vi "FlexMag - 23-03-2023.vi"() -> ()   [LabVIEW 2018] (continued)
            n3949 = local write "CH1_MP_DO"(w6204) -> ()
            n3950 = local write "CH1_TP_BV_DO"(w6207) -> ()
            n3951 = local write "CH1_BG_BV_DO"(w6206) -> ()
            n3952 = local write "CH1_CC_DO"(w6205) -> ()
            n3953 = local write "CH1_Trns_BP_Left_DO"(w6213) -> ()
            n3954 = local write "CH1_SRV1_Piston_For_DO"(w6216) -> ()
            n3955 = local write "CH1_SRV1_Piston_Back_DO"(w6215) -> ()
            n3956 = local write "CH1_WFC_DO"(w6214) -> ()
            n3957 = local read "CH1_PetCool_Down_DI"() -> (w6212:bool)
            n3958 = local read "CH1_Trns_Gv_Open_DI"() -> (w6208:bool)
            n3959 = local read "CH1_Trns_Gv_Close_DI"() -> (w6209:bool)
            n3960 = local read "CH1_Cst_Fix_Down_DI"() -> (w6210:bool)
            n3961 = local read "CH1_PetCool_Up_DI"() -> (w6211:bool)
            n3962 = local read "CH1_TGV_Control_DI"() -> (w6217:bool)
            n3963 = local write "CH1_Trns_Gv_Open_DO"(w6208) -> ()
            n3964 = local write "CH1_Trns_Gv_Close_DO"(w6209) -> ()
            n3965 = local write "CH1_Cst_Fix_DO"(w6210) -> ()
            n3966 = local write "CH1_PetCool_Up_DO"(w6211) -> ()
            n3967 = local write "CH1_PetCool_Down_DO"(w6212) -> ()
            n3968 = local write "CH1_TGV_Control_DO"(w6217) -> ()
          }
        }
      }
      frame #3 {
        # "CH1 DO 1&2"
        n3969 = local read "CH1 I/O Loading"() -> (w6232:bool)
        n3970 = case shown="False" w6232 {
          tunnel: [w6255 w6265] -> w6233
          tunnel: ["CH1_PL_VBV_DO" w6262] -> w6220
          tunnel: ["CH1_CH_VBV_DO" w6262] -> w6219
          frame False {
            n3971 = Build Array("CH1_MP_DO", "CH1_TP_BV_DO", "CH1_BG_BV_DO", "CH1_CH_VBV_DO", "CH1_CH_ATM_DO", "CH1_PL_VBV_DO", "CH1_PL_ATM_DO", "CH1_CC_DO") -> (w6255:bool[])
          }
          frame True {
            w6262 = FALSE
            w6263 = FALSE
            n3972 = local read "CH1_MP_DI"() -> (w6264:bool)
            n3973 = local read "CH1_TP_BV_DI"() -> (w6267:bool)
            n3974 = local read "CH1_BG_BV_DI"() -> (w6268:bool)
            n3975 = local read "CH1_CC_DI"() -> (w6266:bool)
            n3976 = Build Array(w6264, w6267, w6268, w6263, w6263, w6263, w6262, w6266) -> (w6265:bool[])
          }
        }
        "CH1_CH_VBV_DI" <- w6219
        "CH1_PL_VBV_DI" <- w6220
        n3977 = call "MB Serial Master Query Write Multiple Coils (poly).vi"("VISA resource name"=w6224, "Starting Address"=u16 320, "Coils"=w6233, "error in"=w6223, "Serial Parameters"=T15 {"Mode"=enum."RTU", "Slave Address"=1}) -> ("VISA resource name out"=w6229:refnum<visa-resource-name>, "error out"=w6225:errorcluster)  [unwired: 12 in, 1 out]
        n3978 = local read "CH1 I/O Loading"() -> (w6226:bool)
        n3979 = case shown="False" w6226 {
          tunnel: [w6236 w6248] -> w6227
          tunnel: ["CH1_SoV_Ar_DO" w6244] -> w6218
          frame False {
            n3980 = Build Array("CH1_SoV_Ar_DO", "CH1_Trns_Gv_Open_DO", "CH1_Trns_Gv_Close_DO", "CH1_M2_D4_DO", "CH1_Cst_Fix_DO", "CH1_M2_D6_DO", "CH1_PetCool_Up_DO", "CH1_PetCool_Down_DO") -> (w6236:bool[])
          }
          frame True {
            w6244 = FALSE ("element")
            n3981 = local read "CH1_Trns_Gv_Open_DI"() -> (w6252:bool)
            n3982 = local read "CH1_Trns_Gv_Close_DI"() -> (w6251:bool)
            n3983 = local read "CH1_Cst_Fix_Down_DI"() -> (w6247:bool)
            n3984 = local read "CH1_PetCool_Up_DI"() -> (w6246:bool)
            n3985 = local read "CH1_PetCool_Down_DI"() -> (w6245:bool)
            n3986 = local read "CH1_M2_D4_DI"() -> (w6250:bool)
            n3987 = Build Array(w6244, w6252, w6251, w6250, w6247, FALSE ("element"), w6246, w6245) -> (w6248:bool[])
          }
        }
        "CH1_SoV_Ar_DI" <- w6218
        n3988 = call "MB Serial Master Query Write Multiple Coils (poly).vi"("VISA resource name"=w6229, "Starting Address"=u16 320, "Coils"=w6227, "error in"=w6225, "Serial Parameters"=T15 {"Mode"=enum."RTU", "Slave Address"=2}) -> ("VISA resource name out"=w6221:refnum<visa-resource-name>, "error out"=w6222:errorcluster)  [unwired: 12 in, 1 out]
      }
      frame #4 {
        # "CH1 DO 3&4"
        n3989 = local read "CH1 I/O Loading"() -> (w6281:bool)
        n3990 = case shown="False" w6281 {
          tunnel: [w6296 w6306] -> w6280
          frame False {
            n3991 = Build Array("CH1_SRV1_Piston_For_DO", "CH1_SRV1_Piston_Back_DO", "CH1_M3_D3_DO", "CH1_SRV_Direction_Clockwise_DO", "CH1_M3_D5_DO", "CH1_M3_D6_DO", "CH1_WFC_DO", "CH1_Trns_BP_Left_DO") -> (w6296:bool[])
          }
          frame True {
            w6305 = FALSE ("element")
            n3992 = local read "CH1_Trns_BP_Left_DI"() -> (w6307:bool)
            n3993 = local read "CH1_SRV1_Piston_For_DI"() -> (w6308:bool)
            n3994 = local read "CH1_SRV1_Piston_Back_DI"() -> (w6309:bool)
            n3995 = local read "CH1_M3_D6_DI"() -> (w6310:bool)
            n3996 = local read "CH1_WFC_DI"() -> (w6311:bool)
            n3997 = Build Array(w6308, w6309, w6305, w6305, w6305, w6310, w6311, w6307) -> (w6306:bool[])
          }
        }
        n3998 = call "MB Serial Master Query Write Multiple Coils (poly).vi"("VISA resource name"=w6272, "Starting Address"=u16 320, "Coils"=w6280, "error in"=w6271, "Serial Parameters"=T15 {"Mode"=enum."RTU", "Slave Address"=3}) -> ("VISA resource name out"=w6274:refnum<visa-resource-name>, "error out"=w6273:errorcluster)  [unwired: 12 in, 1 out]
        n3999 = local read "CH1 I/O Loading"() -> (w6278:bool)
        n4000 = case shown="False" w6278 {
          tunnel: [w6283 w6292] -> w6275
          frame False {
            n4001 = Build Array("CH1_LN2_DO", "CH1_M4_D2_DO", "CH1_TGV_Control_DO", "CH1_M4_D4_DO", "CH1_Right_Limit_DO", "CH1_Right_Slow_DO", "CH1_M4_D7_DO", "CH1_M4_D8_DO") -> (w6283:bool[])
          }
          frame True {
            w6293 = FALSE ("element")
            w6294 = FALSE ("element")
            n4002 = local read "CH1_TGV_Control_DI"() -> (w6295:bool)
            n4003 = Build Array(w6294, w6294, w6295, w6293, w6293, w6293, w6293, w6293) -> (w6292:bool[])
          }
        }
        n4004 = call "MB Serial Master Query Write Multiple Coils (poly).vi"("VISA resource name"=w6274, "Starting Address"=u16 320, "Coils"=w6275, "error in"=w6273, "Serial Parameters"=T15 {"Mode"=enum."RTU", "Slave Address"=4}) -> ("VISA resource name out"=w6269:refnum<visa-resource-name>, "error out"=w6270:errorcluster)  [unwired: 12 in, 1 out]
      }
      frame #5 {
        # "CH1 AI&AO"
        n4005 = call "MB Serial Master Query Read Input Registers (poly).vi"("VISA resource name"=w6345, "Starting Address"=u16 704 ("Quantity"), "Quantity"=u16 8, "error in"=w6342, "Serial Parameters"=T15 {"Mode"=enum."RTU", "Slave Address"=5}) -> ("VISA resource name out"=w6343:refnum<visa-resource-name>, "Input Registers"=w6333:u16[], "error out"=w6344:errorcluster)  [unwired: 11 in, 1 out]
        n4006 = Index Array(array=w6333, index #1=0 ("index"), index #2=1 ("index"), index #3=2 ("index"), index #4=3 ("index"), index #5=4 ("index"), index #6=5 ("index"), index #7=6 ("index"), index #8=7 ("index")) -> (element #1=→"CH1_Ai_Pl_Pg":u16, element #2=→"CH1_Ai_Ch_Pg":u16, element #3=→"CH1_Ai_Ch_Cc":u16, element #4=→"CH1_Ai_A4":u16, element #5=→"CH1_Ai_A5":u16, element #6=→"CH1_Ai_A6":u16, element #7=→"CH1_LN2_TK_t":u16, element #8=→"CH1_LN2_TK_b":u16)
        n4007 = Build Array(FALSE, "CH1 MW1 Set", "CH1 MW2 Set", "CH1 AO3 Set", "CH1 AO4 Set") -> (w6317:bool[])
        n4008 = Boolean Array To Number(Boolean array=w6317) -> (number=w6316:u32)
        n4009 = Mantissa & Exponent(0:w6316) -> (2:w6315:dbl)  [unwired: 1 out]
        n4010 = case shown="1" w6315 {
          tunnel: [0.0 ("TC2_Set_Value") "CH1 MW1" "CH1 MW2" "CH1 AO3" "CH1 AO4"] -> w6313
          tunnel: [0 1184 1185 1186 1187] -> w6314
          frame 0, Default {
          }
          frame 1 {
            n4011 = local write "CH1 MW1 Set"(FALSE ("CH1 AO1 Set")) -> ()
          }
          frame 2 {
            n4012 = local write "CH1 MW2 Set"(FALSE ("CH1 AO2 Set")) -> ()
          }
          frame 3 {
            n4013 = local write "CH1 AO3 Set"(FALSE ("CH1 AO3 Set")) -> ()
          }
          frame 4 {
            n4014 = local write "CH1 AO4 Set"(FALSE ("CH1 AO4 Set")) -> ()
          }
        }
        n4015 = Build Array(w6313) -> (w6312:dbl[])
        n4016 = call "MB Serial Master Query Write Multiple Registers (poly).vi"("VISA resource name"=w6343, "Starting Address"=w6314, "Registers"=w6312, "error in"=w6344, "Serial Parameters"=T15 {"Mode"=enum."RTU", "Slave Address"=6}) -> ("VISA resource name out"=w6348:refnum<visa-resource-name>, "error out"=w6347:errorcluster)  [unwired: 12 in, 1 out]
      }
      frame #6 {
      }
      frame #7 {
      }
    }
  }
  n4017 = while {
    tunnel: w119 -> [w6370]
    tunnel: w120 -> [w6369]
    tunnel: [w6365] -> w121
    tunnel: [w6364] -> w122
    i -> [w6366]
    stop <- FALSE stop-if-true
    n4018 = Wait Until Next ms Multiple(millisecond multiple=u32 300) -> ()  [unwired: 1 out]
    n4019 = Less Or Equal?(x=w6366, y=5) -> (x <= y?=→"CH3 I/O Loading":bool)
    n4020 = stacked-sequence {
      seq-local: [w6373 _ _ _ _ _ _ _] -> [_ w6422 _ _ _ _ _ _]
      seq-local: [w6374 _ _ _ _ _ _ _] -> [_ w6421 _ _ _ _ _ _]
      seq-local: [_ w6419 _ _ _ _ _ _] -> [_ _ _ w6488 _ _ _ _]
      seq-local: [_ _ _ w6485 _ _ _ _] -> [_ _ _ _ w6536 _ _ _]
      seq-local: [_ _ _ _ w6534 _ _ _] -> [_ _ _ _ _ w6593 _ _]
      seq-local: [_ _ _ w6486 _ _ _ _] -> [_ _ _ _ w6533 _ _ _]
      seq-local: [_ w6420 _ _ _ _ _ _] -> [_ _ _ w6487 _ _ _ _]
      seq-local: [_ _ _ _ w6535 _ _ _] -> [_ _ _ _ _ w6594 _ _]
      tunnel: w6370 -> [w6376 _ _ _ _ _ _ _]
      tunnel: w6369 -> [w6375 _ _ _ _ _ _ _]
      tunnel: [_ _ _ _ _ w6590 _ _] -> w6365
      tunnel: [_ _ _ _ _ w6589 _ _] -> w6364
      frame #0 {
        # "CH3 DI 1&2"
        n4021 = call "MB Serial Master Query Read Discrete Inputs (poly).vi"("VISA resource name"=w6376, "Starting Address"=u16 0 ("Quantity"), "Quantity"=u16 8, "error in"=w6375, "Serial Parameters"=T15 {"Mode"=enum."RTU", "Slave Address"=1}) -> ("VISA resource name out"=w6409:refnum<visa-resource-name>, "Discrete Inputs"=w6393:bool[], "error out"=w6408:errorcluster)  [unwired: 11 in, 1 out]
        n4022 = Index Array(array=w6393, index #1=0 ("index"), index #2=1 ("index"), index #3=2 ("index"), index #4=3 ("index"), index #5=4 ("index"), index #6=5 ("index"), index #7=6 ("index"), index #8=7 ("index")) -> (element #1=→"CH3_MP_DI":bool, element #2=→"CH3_TP_BV_DI":bool, element #3=→"CH3_BG_BV_DI":bool, element #5=→"CH3_CH_ATM_DI":bool, element #7=→"CH3_PL_ATM_DI":bool, element #8=→"CH3_CC_DI":bool)  [unwired: 2 out]
        n4023 = call "MB Serial Master Query Read Discrete Inputs (poly).vi"("VISA resource name"=w6409, "Starting Address"=u16 0 ("Quantity"), "Quantity"=u16 8, "error in"=w6408, "Serial Parameters"=T15 {"Mode"=enum."RTU", "Slave Address"=2}) -> ("VISA resource name out"=w6373:refnum<visa-resource-name>, "Discrete Inputs"=w6377:bool[], "error out"=w6374:errorcluster)  [unwired: 11 in, 1 out]
        n4024 = Index Array(array=w6377, index #1=0 ("index"), index #2=1 ("index"), index #3=2 ("index"), index #4=3 ("index"), index #5=4 ("index"), index #6=5 ("index"), index #7=6 ("index"), index #8=7 ("index")) -> (element #2=→"CH3_Trns_Gv_Open_DI":bool, element #3=→"CH3_Trns_Gv_Close_DI":bool, element #4=→"CH3_Trns_BP_Right_DI":bool, element #5=→"CH3_Cst_Fix_Up_DI":bool, element #6=→"CH3_Cst_Fix_Down_DI":bool, element #7=→"CH3_PetCool_Up_DI":bool, element #8=→"CH3_PetCool_Down_DI":bool)  [unwired: 1 out]
      }
      frame #1 {
        # "CH3 DI 3&4"
        n4025 = call "MB Serial Master Query Read Discrete Inputs (poly).vi"("VISA resource name"=w6422, "Starting Address"=u16 0 ("Quantity"), "Quantity"=u16 8, "error in"=w6421, "Serial Parameters"=T15 {"Mode"=enum."RTU", "Slave Address"=3}) -> ("VISA resource name out"=w6457:refnum<visa-resource-name>, "Discrete Inputs"=w6440:bool[], "error out"=w6456:errorcluster)  [unwired: 11 in, 1 out]
        n4026 = local read "water bypass"() -> (w6418:bool)
        n4027 = Index Array(array=w6440, index #1=0 ("index"), index #2=1 ("index"), index #3=2 ("index"), index #4=3 ("index"), index #5=4 ("index"), index #6=5 ("index"), index #7=6 ("index"), index #8=7 ("index")) -> (element #1=→"CH3_SRV1_Piston_For_DI":bool, element #2=→"CH3_SRV1_Piston_Back_DI":bool, element #3=→"CH3_SRV_Start_Stop_DI":bool, element #4=→"CH3_SRV_Left_Direction_DI3":bool, element #5=→"CH3_SRV2_COUNTER_DI":bool, element #6=→"CH3_M3_D6_DI":bool, element #7=w6416:bool, element #8=→"CH3_Trns_BP_Left_DI":bool)
        n4028 = case shown="True" w6418 {
          tunnel: w6416 -> [w6464 _]
          tunnel: [w6464 w6465] -> w6417
          frame False {
          }
          frame True {
            n4029 = local read "CH3_WFC_DO"() -> (w6465:bool)
          }
        }
        "CH3_WFC_DI" <- w6417
        n4030 = call "MB Serial Master Query Read Discrete Inputs (poly).vi"("VISA resource name"=w6457, "Starting Address"=u16 0 ("Quantity"), "Quantity"=u16 8, "error in"=w6456, "Serial Parameters"=T15 {"Mode"=enum."RTU", "Slave Address"=4}) -> ("VISA resource name out"=w6419:refnum<visa-resource-name>, "Discrete Inputs"=w6423:bool[], "error out"=w6420:errorcluster)  [unwired: 11 in, 1 out]
        n4031 = Index Array(array=w6423, index #1=0 ("index"), index #2=1 ("index"), index #3=2 ("index"), index #4=3 ("index"), index #5=4 ("index"), index #6=5 ("index"), index #7=6 ("index"), index #8=7 ("index")) -> (element #1=→"CH3_Air_Pressure_DI":bool, element #2=→"CH3_DS_DI":bool, element #3=→"CH3_TGV_Control_DI":bool, element #4=→"CH3_Trns_Interlock_DI":bool, element #5=→"CH3_Right_Limit_DI":bool, element #6=→"CH3_Right_Slow_DI":bool, element #7=→"CH3_Left_Slow_DI":bool, element #8=→"CH3_Left_Limit_DI":bool)
      }
      frame #2 {
        n4032 = local read "CH3 I/O Loading"() -> (w6466:bool)
        n4033 = case shown="True" w6466 {
          frame False {
          }
          frame True {
            n4034 = local read "CH3_SRV1_Piston_Back_DI"() -> (w6470:bool)
            n4035 = local read "CH3_SRV1_Piston_For_DI"() -> (w6471:bool)
            n4036 = local read "CH3_Trns_BP_Left_DI"() -> (w6468:bool)
            n4037 = local read "CH3_BG_BV_DI"() -> (w6473:bool)
            n4038 = local read "CH3_TP_BV_DI"() -> (w6474:bool)
            n4039 = local read "CH3_WFC_DI"() -> (w6469:bool)
            n4040 = local read "CH3_MP_DI"() -> (w6475:bool)
            n4041 = local read "CH3_CC_DI"() -> (w6472:bool)
            n4042 = local write "CH3_MP_DO"(w6475) -> ()
            n4043 = local write "CH3_TP_BV_DO"(w6474) -> ()
            n4044 = local write "CH3_BG_BV_DO"(w6473) -> ()
            n4045 = local write "CH3_CC_DO"(w6472) -> ()
            n4046 = local write "CH3_Trns_BP_Left_DO"(w6468) -> ()
            n4047 = local write "CH3_SRV1_Piston_For_DO"(w6471) -> ()
            n4048 = local write "CH3_SRV1_Piston_Back_DO"(w6470) -> ()
            n4049 = local write "CH3_WFC_DO"(w6469) -> ()
            n4050 = local read "CH3_PetCool_Down_DI"() -> (w6481:bool)
            n4051 = local read "CH3_Trns_Gv_Open_DI"() -> (w6476:bool)
            n4052 = local read "CH3_Trns_Gv_Close_DI"() -> (w6477:bool)
            n4053 = local read "CH3_Cst_Fix_Down_DI"() -> (w6479:bool)
            n4054 = local read "CH3_Trns_BP_Right_DI"() -> (w6478:bool)
            n4055 = local read "CH3_PetCool_Up_DI"() -> (w6480:bool)
            n4056 = local read "CH3_TGV_Control_DI"() -> (w6467:bool)
            n4057 = local write "CH3_Trns_BP_Right_DO"(w6478) -> ()
            n4058 = local write "CH3_Trns_GV_Open_DO"(w6476) -> ()
            n4059 = local write "CH3_Trns_GV_Close_DO"(w6477) -> ()
            n4060 = local write "CH3_Cst_Fix_DO"(w6479) -> ()
            n4061 = local write "CH3_PetCool_Up_DO"(w6480) -> ()
            n4062 = local write "CH3_PetCool_Down_DO"(w6481) -> ()
            n4063 = local write "CH3_TGV_Control_DO"(w6467) -> ()
          }
        }
      }
      frame #3 {
        # "CH3 DO 1&2"
        n4064 = local read "CH3 I/O Loading"() -> (w6490:bool)
        n4065 = case shown="False" w6490 {
          tunnel: [w6519 w6532] -> w6492
          tunnel: ["CH3_PL_VBV_DO" w6527] -> w6484
          tunnel: ["CH3_CH_VBV_DO" w6527] -> w6483
          frame False {
            n4066 = Build Array("CH3_MP_DO", "CH3_TP_BV_DO", "CH3_BG_BV_DO", "CH3_CH_VBV_DO", "CH3_CH_ATM_DO", "CH3_PL_VBV_DO", "CH3_PL_ATM_DO", "CH3_CC_DO") -> (w6519:bool[])
          }
          frame True {
            w6527 = FALSE
            w6526 = FALSE
            n4067 = local read "CH3_CC_DI"() -> (w6528:bool)
            n4068 = local read "CH3_BG_BV_DI"() -> (w6529:bool)
            n4069 = local read "CH3_TP_BV_DI"() -> (w6531:bool)
            n4070 = local read "CH3_MP_DI"() -> (w6530:bool)
            n4071 = Build Array(w6530, w6531, w6529, w6526, w6526, w6526, w6527, w6528) -> (w6532:bool[])
          }
        }
        "CH3_CH_VBV_DI" <- w6483
        "CH3_PL_VBV_DI" <- w6484
        n4072 = call "MB Serial Master Query Write Multiple Coils (poly).vi"("VISA resource name"=w6488, "Starting Address"=u16 320, "Coils"=w6492, "error in"=w6487, "Serial Parameters"=T15 {"Mode"=enum."RTU", "Slave Address"=1}) -> ("VISA resource name out"=w6494:refnum<visa-resource-name>, "error out"=w6493:errorcluster)  [unwired: 12 in, 1 out]
        n4073 = local read "CH3 I/O Loading"() -> (w6489:bool)
        n4074 = case shown="False" w6489 {
          tunnel: [w6500 w6516] -> w6491
          tunnel: ["CH3_SoV_Ar_DO" w6508] -> w6482
          frame False {
            n4075 = Build Array("CH3_SoV_Ar_DO", "CH3_Trns_GV_Open_DO", "CH3_Trns_GV_Close_DO", "CH3_Trns_BP_Right_DO", "CH3_Cst_Fix_DO", "CH3_M2_D6_DO", "CH3_PetCool_Up_DO", "CH3_PetCool_Down_DO") -> (w6500:bool[])
          }
          frame True {
            w6508 = FALSE
            n4076 = local read "CH3_PetCool_Down_DI"() -> (w6514:bool)
            n4077 = local read "CH3_Trns_Gv_Open_DI"() -> (w6515:bool)
            n4078 = local read "CH3_Trns_Gv_Close_DI"() -> (w6510:bool)
            n4079 = local read "CH3_Trns_BP_Right_DI"() -> (w6511:bool)
            n4080 = local read "CH3_Cst_Fix_Down_DI"() -> (w6512:bool)
            n4081 = local read "CH3_PetCool_Up_DI"() -> (w6513:bool)
            n4082 = Build Array(w6508, w6515, w6510, w6511, w6512, FALSE ("element"), w6513, w6514) -> (w6516:bool[])
          }
        }
        "CH3_SoV_Ar_DI" <- w6482
        n4083 = call "MB Serial Master Query Write Multiple Coils (poly).vi"("VISA resource name"=w6494, "Starting Address"=u16 320, "Coils"=w6491, "error in"=w6493, "Serial Parameters"=T15 {"Mode"=enum."RTU", "Slave Address"=2}) -> ("VISA resource name out"=w6485:refnum<visa-resource-name>, "error out"=w6486:errorcluster)  [unwired: 12 in, 1 out]
      }
      frame #4 {
        # "CH3 DO 3&4"
        n4084 = local read "CH3 I/O Loading"() -> (w6538:bool)
        n4085 = case shown="False" w6538 {
          tunnel: [w6560 w6575] -> w6539
          frame False {
            n4086 = Build Array("CH3_SRV1_Piston_For_DO", "CH3_SRV1_Piston_Back_DO", "CH3_M3_D3_DO", "CH3_SRV_Direction_Clockwise_DO", "CH3_M3_D5_DO", "CH3_M3_D6_DO", "CH3_WFC_DO", "CH3_Trns_BP_Left_DO") -> (w6560:bool[])
          }
          frame True {
            w6569 = FALSE
            n4087 = local read "CH3_SRV1_Piston_Back_DI"() -> (w6573:bool)
            n4088 = local read "CH3_SRV1_Piston_For_DI"() -> (w6574:bool)
            n4089 = local read "CH3_Trns_BP_Left_DI"() -> (w6570:bool)
            n4090 = local read "CH3_M3_D6_DI"() -> (w6572:bool)
            n4091 = local read "CH3_WFC_DI"() -> (w6571:bool)
            n4092 = Build Array(w6574, w6573, w6569, w6569, w6569, w6572, w6571, w6570) -> (w6575:bool[])
          }
        }
        n4093 = call "MB Serial Master Query Write Multiple Coils (poly).vi"("VISA resource name"=w6536, "Starting Address"=u16 320, "Coils"=w6539, "error in"=w6533, "Serial Parameters"=T15 {"Mode"=enum."RTU", "Slave Address"=3}) -> ("VISA resource name out"=w6542:refnum<visa-resource-name>, "error out"=w6541:errorcluster)  [unwired: 12 in, 1 out]
        n4094 = local read "CH3 I/O Loading"() -> (w6537:bool)
        n4095 = case shown="False" w6537 {
          tunnel: [w6547 w6557] -> w6540
          frame False {
            n4096 = Build Array("CH3_LN2_DO", "CH3_M4_D2_DO", "CH3_TGV_Control_DO", "CH3_M4_D4_DO", "CH3_Right_Limit_DO", "CH3_Right_Slow_DO", "CH3_Left_Slow_DO", "CH3_Left_Limit_DO") -> (w6547:bool[])
          }
          frame True {
            w6559 = FALSE
            w6558 = FALSE
            n4097 = local read "CH3_TGV_Control_DI"() -> (w6556:bool)
            n4098 = Build Array(w6558, w6558, w6556, w6559, w6559, w6559, w6559, w6559) -> (w6557:bool[])
          }
        }
        n4099 = call "MB Serial Master Query Write Multiple Coils (poly).vi"("VISA resource name"=w6542, "Starting Address"=u16 320, "Coils"=w6540, "error in"=w6541, "Serial Parameters"=T15 {"Mode"=enum."RTU", "Slave Address"=4}) -> ("VISA resource name out"=w6535:refnum<visa-resource-name>, "error out"=w6534:errorcluster)  [unwired: 12 in, 1 out]
      }
      frame #5 {
        # "CH3 AI&AO"
        n4100 = call "MB Serial Master Query Read Input Registers (poly).vi"("VISA resource name"=w6594, "Starting Address"=u16 704, "Quantity"=u16 8, "error in"=w6593, "Serial Parameters"=T15 {"Mode"=enum."RTU", "Slave Address"=5}) -> ("VISA resource name out"=w6592:refnum<visa-resource-name>, "Input Registers"=w6605:u16[], "error out"=w6591:errorcluster)  [unwired: 11 in, 1 out]
        n4101 = Index Array(array=w6605, index #1=0 ("index"), index #2=1 ("index"), index #3=2 ("index"), index #4=3 ("index"), index #5=4 ("index"), index #6=5 ("index"), index #7=6 ("index"), index #8=7 ("index")) -> (element #1=→"CH3_Ai_Pl_Pg":u16, element #2=→"CH3_Ai_Ch_Pg":u16, element #3=→"CH3_Ai_Ch_Cc":u16, element #4=→"MFC_Ar_Read_value":u16, element #5=→"CH3_Ai_A5":u16, element #6=→"CH3_Ai_A6":u16, element #7=→"CH3_LN2_TK_t":u16, element #8=→"CH3_LN2_TK_b":u16)
        n4102 = Build Array(FALSE, "CH3 AO1 Set", "CH3 AO2 Set", "CH3 AO3 Set", "MFC_Ar_Set") -> (w6581:bool[])
        n4103 = Boolean Array To Number(Boolean array=w6581) -> (number=w6580:u32)
        n4104 = Mantissa & Exponent(0:w6580) -> (2:w6579:dbl)  [unwired: 1 out]
        n4105 = case shown="4" w6579 {
          tunnel: [0.0 ("TC2_Set_Value") "CH3 AO1" "CH3 AO2" "CH3 AO3" w6628] -> w6577
          tunnel: [0 1184 1185 1186 1187] -> w6578
          frame 0, Default {
          }
          frame 1 {
            n4106 = local write "CH3 AO1 Set"(FALSE ("CH1 AO1 Set")) -> ()
          }
          frame 2 {
            n4107 = local write "CH3 AO2 Set"(FALSE ("CH1 AO2 Set")) -> ()
          }
          frame 3 {
            n4108 = local write "CH3 AO3 Set"(FALSE ("CH1 AO3 Set")) -> ()
          }
          frame 4 {
            n4109 = local write "MFC_Ar_Set"(FALSE ("CH2 AO4 Set")) -> ()
            n4110 = Divide(x=2048.0, y=200.0) -> (x/y=w6630:dbl)
            n4111 = Multiply(x="MFC_Ar_Set_value", y=w6630) -> (x*y=w6627:dbl)
            n4112 = In Range and Coerce(upper limit=2048.0, x=w6627, lower limit=0.0) -> (coerced(x)=w6628:dbl)  [unwired: 1 out]
          }
        }
        n4113 = Build Array(w6577) -> (w6576:dbl[])
        n4114 = call "MB Serial Master Query Write Multiple Registers (poly).vi"("VISA resource name"=w6592, "Starting Address"=w6578, "Registers"=w6576, "error in"=w6591, "Serial Parameters"=T15 {"Mode"=enum."RTU", "Slave Address"=6}) -> ("VISA resource name out"=w6590:refnum<visa-resource-name>, "error out"=w6589:errorcluster)  [unwired: 12 in, 1 out]
      }
      frame #6 {
      }
      frame #7 {
      }
    }
  }
  n4115 = while {
    tunnel: w144 -> [w6641]
    tunnel: w143 -> [w6640]
    tunnel: [w6639] -> w142
    tunnel: [w6638] -> w141
    i -> [w6637]
    stop <- FALSE stop-if-true
    n4116 = Wait Until Next ms Multiple(millisecond multiple=u32 300) -> ()  [unwired: 1 out]
    n4117 = Less Or Equal?(x=w6637, y=5) -> (x <= y?=→"Center I/O Loading":bool)
    n4118 = stacked-sequence {
      seq-local: [w6647 _ _] -> [_ w6692 _]
      seq-local: [w6646 _ _] -> [_ w6691 _]
      seq-local: [_ w6693 _] -> [_ _ w6745]
      seq-local: [_ w6690 _] -> [_ _ w6744]
      tunnel: w6641 -> [w6648 _ _]
      tunnel: w6640 -> [w6645 _ _]
      tunnel: [_ _ w6743] -> w6639
      tunnel: [_ _ w6742] -> w6638
      frame #0 {
        # "Digital Inputs"
        n4119 = call "MB Serial Master Query Read Discrete Inputs (poly).vi"("VISA resource name"=w6648, "Starting Address"=u16 0 ("Quantity"), "Quantity"=u16 8, "error in"=w6645, "Serial Parameters"=T15 {"Mode"=enum."RTU", "Slave Address"=1}) -> ("VISA resource name out"=w6667:refnum<visa-resource-name>, "Discrete Inputs"=w6683:bool[], "error out"=w6666:errorcluster)  [unwired: 11 in, 1 out]
        n4120 = Index Array(array=w6683, index #1=0 ("index"), index #2=1 ("index"), index #3=2 ("index"), index #4=3 ("index"), index #5=4 ("index"), index #6=5 ("index"), index #7=6 ("index"), index #8=7 ("index")) -> (element #1=→"Casette_Servo_Start/Stop DI":bool, element #2=→"Casette_Servo_Left_Direction DI":bool, element #3=→"Tension_Controllers_Start/Stop DI":bool, element #4=→"Cnt_Right_Limit DI":bool, element #5=→"Cnt_Right_Slow DI":bool, element #6=→"Cnt_Left_Slow DI":bool, element #7=→"Cnt_Left_Limit DI":bool, element #8=→"WFC DI":bool)
        n4121 = call "MB Serial Master Query Read Discrete Inputs (poly).vi"("VISA resource name"=w6667, "Starting Address"=u16 0 ("Quantity"), "Quantity"=u16 8, "error in"=w6666, "Serial Parameters"=T15 {"Mode"=enum."RTU", "Slave Address"=2}) -> ("VISA resource name out"=w6647:refnum<visa-resource-name>, "Discrete Inputs"=w6657:bool[], "error out"=w6646:errorcluster)  [unwired: 11 in, 1 out]
        n4122 = Index Array(array=w6657, index #1=0 ("index"), index #2=1 ("index"), index #3=2 ("index"), index #4=3 ("index"), index #5=4 ("index"), index #6=5 ("index"), index #7=6 ("index"), index #8=7 ("index")) -> (element #1=→"DCPS_ SW1 DI":bool, element #2=→"DCPS_ SW2 DI":bool, element #3=→"DCPS_ SW3 DI":bool, element #4=→"DCPS_ SW4 DI":bool, element #5=→"MW1 DI":bool, element #6=→"MW2 DI":bool, element #7=→"Center_2 DI7":bool, element #8=→"Center_2 DI8":bool)
      }
      frame #1 {
        # "Digital Outputs"
        n4123 = local read "Center I/O Loading"() -> (w6695:bool)
        n4124 = case shown="False" w6695 {
          tunnel: [w6722 w6731] -> w6702
          frame False {
            n4125 = Build Array("Casette_Servo_Start/Stop DO", "Casette_Servo_Left_Direction DO", "Tension_Controllers_Start/Stop DO", "Cnt_Right_Limit DO", "Cnt_Right_Slow DO", "Cnt_Left_Slow DO", "Cnt_Left_Limit DO", "Buzzer DO") -> (w6722:bool[])
          }
          frame True {
            n4126 = local read "Tension_Controllers_Start/Stop DI"() -> (w6737:bool)
            n4127 = local read "Casette_Servo_Left_Direction DI"() -> (w6738:bool)
            n4128 = local read "Casette_Servo_Start/Stop DI"() -> (w6739:bool)
            n4129 = local read "Cnt_Right_Limit DI"() -> (w6736:bool)
            n4130 = local read "Cnt_Right_Slow DI"() -> (w6735:bool)
            n4131 = local read "Cnt_Left_Slow DI"() -> (w6734:bool)
            n4132 = local read "Cnt_Left_Limit DI"() -> (w6733:bool)
            n4133 = Build Array(w6739, w6738, w6737, w6736, w6735, w6734, w6733, FALSE ("element")) -> (w6731:bool[])
          }
        }
        n4134 = call "MB Serial Master Query Write Multiple Coils (poly).vi"("VISA resource name"=w6692, "Starting Address"=u16 320, "Coils"=w6702, "error in"=w6691, "Serial Parameters"=T15 {"Mode"=enum."RTU", "Slave Address"=1}) -> ("VISA resource name out"=w6697:refnum<visa-resource-name>, "error out"=w6696:errorcluster)  [unwired: 12 in, 1 out]
        n4135 = local read "Center I/O Loading"() -> (w6694:bool)
        n4136 = case shown="True" w6694 {
          tunnel: [w6712 w6717] -> w6699
          frame False {
            n4137 = Build Array("DCPS_ SW1 DO", "DCPS_ SW2 DO", "DCPS_ SW3  DO", "DCPS_ SW4 DO", "Center_2 DO5", "Center_2 DO6", "Center_2 DO7", "Center_2 DO8") -> (w6712:bool[])
          }
          frame True {
            n4138 = local read "DCPS_ SW3 DI"() -> (w6719:bool)
            n4139 = local read "DCPS_ SW2 DI"() -> (w6720:bool)
            n4140 = local read "DCPS_ SW4 DI"() -> (w6718:bool)
            n4141 = local read "DCPS_ SW1 DI"() -> (w6721:bool)
            n4142 = Build Array(w6721, w6720, w6719, w6718, FALSE ("element"), FALSE ("element"), FALSE ("element"), FALSE ("element")) -> (w6717:bool[])
          }
        }
        n4143 = call "MB Serial Master Query Write Multiple Coils (poly).vi"("VISA resource name"=w6697, "Starting Address"=u16 320, "Coils"=w6699, "error in"=w6696, "Serial Parameters"=T15 {"Mode"=enum."RTU", "Slave Address"=2}) -> ("VISA resource name out"=w6693:refnum<visa-resource-name>, "error out"=w6690:errorcluster)  [unwired: 12 in, 1 out]
      }
      frame #2 {
        # "Analog Outputs"
        n4144 = Build Array(FALSE, "Center AO1 Set", "Cassette_Servo_Speed Set", "TC1 Set moxa", "TC2 Set moxa") -> (w6754:bool[])
        n4145 = Boolean Array To Number(Boolean array=w6754) -> (number=w6755:u32)
        n4146 = Mantissa & Exponent(0:w6755) -> (2:w6749:dbl)  [unwired: 1 out]
        n4147 = case shown="2" w6749 {
          tunnel: [0.0 ("TC2_Set_Value") "Center AO1" "Cassette_Servo_Speed AO" w6764 w6772] -> w6748
          tunnel: [0 1184 1185 1186 1187] -> w6746
          frame 0, Default {
          }
          frame 1 {
            n4148 = local write "Center AO1 Set"(FALSE ("Center AO1 Set")) -> ()
          }
          frame 2 {
            n4149 = local write "Cassette_Servo_Speed Set"(FALSE ("Center AO2 Set")) -> ()
          }
          frame 3 {
            n4150 = local write "TC1 Set moxa"(FALSE ("TC1 Set")) -> ()
            n4151 = Divide(x=4096.0, y=10.0) -> (x/y=w6768:dbl)
            n4152 = Multiply(x=w6768, y="TC1_Set_Value_Moxa") -> (x*y=w6764:dbl)
          }
          frame 4 {
            n4153 = local write "TC2 Set moxa"(FALSE ("TC2 Set")) -> ()
            n4154 = Divide(x=4096.0, y=10.0) -> (x/y=w6775:dbl)
            n4155 = Multiply(x=w6775, y="TC2_Set_Value_Moxa") -> (x*y=w6772:dbl)
          }
        }
        n4156 = Build Array(w6748) -> (w6747:dbl[])
        n4157 = call "MB Serial Master Query Write Multiple Registers (poly).vi"("VISA resource name"=w6745, "Starting Address"=w6746, "Registers"=w6747, "error in"=w6744, "Serial Parameters"=T15 {"Mode"=enum."RTU", "Slave Address"=3}) -> ("VISA resource name out"=w6743:refnum<visa-resource-name>, "error out"=w6742:errorcluster)  [unwired: 12 in, 1 out]
      }
    }
  }
  n4158 = while {
    tunnel: w126 -> [w6784]
    tunnel: w125 -> [w6783]
    tunnel: [w6779] -> w124
    tunnel: [w6778] -> w123
    i -> [w6780]
    stop <- FALSE stop-if-true
    n4159 = Wait Until Next ms Multiple(millisecond multiple=u32 300) -> ()  [unwired: 1 out]
    n4160 = Less Or Equal?(x=w6780, y=5) -> (x <= y?=→"CH2 I/O Loading":bool)
    n4161 = stacked-sequence {
      seq-local: [w6789 _ _ _ _ _ _ _] -> [_ w6836 _ _ _ _ _ _]
      seq-local: [w6788 _ _ _ _ _ _ _] -> [_ w6834 _ _ _ _ _ _]
      seq-local: [_ w6835 _ _ _ _ _ _] -> [_ _ _ w6902 _ _ _ _]
      seq-local: [_ _ _ w6899 _ _ _ _] -> [_ _ _ _ w6951 _ _ _]
      seq-local: [_ _ _ _ w6949 _ _ _] -> [_ _ _ _ _ w7009 _ _]
      seq-local: [_ _ _ w6900 _ _ _ _] -> [_ _ _ _ w6950 _ _ _]
      seq-local: [_ w6833 _ _ _ _ _ _] -> [_ _ _ w6901 _ _ _ _]
      seq-local: [_ _ _ _ w6948 _ _ _] -> [_ _ _ _ _ w7010 _ _]
      tunnel: w6784 -> [w6790 _ _ _ _ _ _ _]
      tunnel: w6783 -> [w6787 _ _ _ _ _ _ _]
      tunnel: [_ _ _ _ _ w7006 _ _] -> w6779
      tunnel: [_ _ _ _ _ w7005 _ _] -> w6778
      frame #0 {
        # "CH2 DI 1&2"
        n4162 = call "MB Serial Master Query Read Discrete Inputs (poly).vi"("VISA resource name"=w6790, "Starting Address"=u16 0 ("Quantity"), "Quantity"=u16 8, "error in"=w6787, "Serial Parameters"=T15 {"Mode"=enum."RTU", "Slave Address"=1}) -> ("VISA resource name out"=w6823:refnum<visa-resource-name>, "Discrete Inputs"=w6807:bool[], "error out"=w6822:errorcluster)  [unwired: 11 in, 1 out]
        n4163 = Index Array(array=w6807, index #1=0 ("index"), index #2=1 ("index"), index #3=2 ("index"), index #4=3 ("index"), index #5=4 ("index"), index #6=5 ("index"), index #7=6 ("index"), index #8=7 ("index")) -> (element #1=→"CH2_MP_DI":bool, element #2=→"CH2_TP_BV_DI":bool, element #3=→"CH2_BG_BV_DI":bool, element #5=→"CH2_CH_ATM_DI":bool, element #7=→"CH2_PL_ATM_DI":bool, element #8=→"CH2_CC_DI":bool)  [unwired: 2 out]
        n4164 = call "MB Serial Master Query Read Discrete Inputs (poly).vi"("VISA resource name"=w6823, "Starting Address"=u16 0 ("Quantity"), "Quantity"=u16 8, "error in"=w6822, "Serial Parameters"=T15 {"Mode"=enum."RTU", "Slave Address"=2}) -> ("VISA resource name out"=w6789:refnum<visa-resource-name>, "Discrete Inputs"=w6791:bool[], "error out"=w6788:errorcluster)  [unwired: 11 in, 1 out]
        n4165 = Index Array(array=w6791, index #1=0 ("index"), index #2=1 ("index"), index #3=2 ("index"), index #4=3 ("index"), index #5=4 ("index"), index #6=5 ("index"), index #7=6 ("index"), index #8=7 ("index")) -> (element #2=→"CH2_Trns_Gv_Open_DI":bool, element #3=→"CH2_Trns_Gv_Close_DI":bool, element #4=→"CH2_Trns_BP_Right_DI":bool, element #5=→"CH2_Cst_Fix_Up_DI":bool, element #6=→"CH2_Cst_Fix_Down_DI":bool, element #7=→"CH2_PetCool_Up_DI":bool, element #8=→"CH2_PetCool_Down_DI":bool)  [unwired: 1 out]
      }
      frame #1 {
        n4166 = call "MB Serial Master Query Read Discrete Inputs (poly).vi"("VISA resource name"=w6836, "Starting Address"=u16 0 ("Quantity"), "Quantity"=u16 8, "error in"=w6834, "Serial Parameters"=T15 {"Mode"=enum."RTU", "Slave Address"=3}) -> ("VISA resource name out"=w6871:refnum<visa-resource-name>, "Discrete Inputs"=w6837:bool[], "error out"=w6870:errorcluster)  [unwired: 11 in, 1 out]
        n4167 = local read "water bypass"() -> (w6832:bool)
        n4168 = Index Array(array=w6837, index #1=0 ("index"), index #2=1 ("index"), index #3=2 ("index"), index #4=3 ("index"), index #5=4 ("index"), index #6=5 ("index"), index #7=6 ("index"), index #8=7 ("index")) -> (element #1=→"CH2_SRV1_Piston_For_DI":bool, element #2=→"CH2_SRV1_Piston_Back_DI":bool, element #3=→"CH2_SRV_Start_Stop_DI":bool, element #4=→"CH2_SRV_Left_Direction_DI":bool, element #5=→"CH2_SRV2_COUNTER_DI":bool, element #6=→"CH2_M3_D6_DI":bool, element #7=w6831:bool, element #8=→"CH2_Trns_BP_Left_DI":bool)
        n4169 = case shown="True" w6832 {
          tunnel: w6831 -> [w6878 _]
          tunnel: [w6878 w6879] -> w6830
          frame False {
          }
          frame True {
            n4170 = local read "CH2_WFC_DO"() -> (w6879:bool)
          }
        }
        "CH2_WFC_DI" <- w6830
        n4171 = call "MB Serial Master Query Read Discrete Inputs (poly).vi"("VISA resource name"=w6871, "Starting Address"=u16 0 ("Quantity"), "Quantity"=u16 8, "error in"=w6870, "Serial Parameters"=T15 {"Mode"=enum."RTU", "Slave Address"=4}) -> ("VISA resource name out"=w6835:refnum<visa-resource-name>, "Discrete Inputs"=w6853:bool[], "error out"=w6833:errorcluster)  [unwired: 11 in, 1 out]
        n4172 = Index Array(array=w6853, index #1=0 ("index"), index #2=1 ("index"), index #3=2 ("index"), index #4=3 ("index"), index #5=4 ("index"), index #6=5 ("index"), index #7=6 ("index"), index #8=7 ("index")) -> (element #1=→"CH2_Air_Pressure_DI":bool, element #2=→"CH2_DS_DI":bool, element #3=→"CH2_TGV_Control_DI":bool, element #4=→"CH2_Trns_Interlock_DI":bool, element #5=→"CH2_Right_Limit_DI":bool, element #6=→"CH2_Right_Slow_DI":bool, element #7=→"CH2_Left_Slow_DI":bool, element #8=→"CH2_Left_Limit_DI":bool)
      }
      frame #2 {
        n4173 = local read "CH2 I/O Loading"() -> (w6880:bool)
        n4174 = case shown="True" w6880 {
          frame False {
          }
          frame True {
            n4175 = local read "CH2_BG_BV_DI"() -> (w6893:bool)
            n4176 = local read "CH2_TP_BV_DI"() -> (w6894:bool)
            n4177 = local read "CH2_SRV1_Piston_Back_DI"() -> (w6884:bool)
            n4178 = local read "CH2_SRV1_Piston_For_DI"() -> (w6885:bool)
            n4179 = local read "CH2_MP_DI"() -> (w6895:bool)
            n4180 = local read "CH2_CC_DI"() -> (w6892:bool)
            n4181 = local read "CH2_Trns_BP_Left_DI"() -> (w6883:bool)
            n4182 = local read "CH2_WFC_DI"() -> (w6882:bool)
            n4183 = local write "CH2_MP_DO"(w6895) -> ()
            n4184 = local write "CH2_TP_BV_DO"(w6894) -> ()
            n4185 = local write "CH2_BG_BV_DO"(w6893) -> ()
            n4186 = local write "CH2_CC_DO"(w6892) -> ()
            n4187 = local write "CH2_Trns_BP_Left_DO"(w6883) -> ()
            n4188 = local write "CH2_SRV1_Piston_For_DO"(w6885) -> ()
            n4189 = local write "CH2_SRV1_Piston_Back_DO"(w6884) -> ()
            n4190 = local write "CH2_WFC_DO"(w6882) -> ()
            n4191 = local read "CH2_PetCool_Down_DI"() -> (w6886:bool)
            n4192 = local read "CH2_Trns_Gv_Open_DI"() -> (w6891:bool)
            n4193 = local read "CH2_Trns_Gv_Close_DI"() -> (w6890:bool)
            n4194 = local read "CH2_Cst_Fix_Down_DI"() -> (w6888:bool)
            n4195 = local read "CH2_Trns_BP_Right_DI"() -> (w6889:bool)
            n4196 = local read "CH2_PetCool_Up_DI"() -> (w6887:bool)
            n4197 = local read "CH2_TGV_Control_DI"() -> (w6881:bool)
            n4198 = local write "CH2_Trns_BP_Right_DO"(w6889) -> ()
            n4199 = local write "CH2_Trns_GV_Open_DO"(w6891) -> ()
            n4200 = local write "CH2_Trns_GV_Close_DO"(w6890) -> ()
            n4201 = local write "CH2_Cst_Fix_DO"(w6888) -> ()
            n4202 = local write "CH2_PetCool_Up_DO"(w6887) -> ()
            n4203 = local write "CH2_PetCool_Down_DO"(w6886) -> ()
            n4204 = local write "CH2_TGV_Control_DO"(w6881) -> ()
          }
        }
      }
      frame #3 {
        # "CH2 DO 1&2"
        n4205 = local read "CH2 I/O Loading"() -> (w6904:bool)
        n4206 = case shown="False" w6904 {
          tunnel: [w6933 w6943] -> w6906
          tunnel: ["CH2_CH_VBV_DO" w6940] -> w6897
          tunnel: ["CH2_PL_VBV_DO" w6940] -> w6896
          frame False {
            n4207 = Build Array("CH2_MP_DO", "CH2_TP_BV_DO", "CH2_BG_BV_DO", "CH2_CH_VBV_DO", "CH2_CH_ATM_DO", "CH2_PL_VBV_DO", "CH2_PL_ATM_DO", "CH2_CC_DO") -> (w6933:bool[])
          }
          frame True {
            w6940 = FALSE
            w6941 = FALSE
            n4208 = local read "CH2_BG_BV_DI"() -> (w6945:bool)
            n4209 = local read "CH2_TP_BV_DI"() -> (w6946:bool)
            n4210 = local read "CH2_CC_DI"() -> (w6944:bool)
            n4211 = local read "CH2_MP_DI"() -> (w6947:bool)
            n4212 = Build Array(w6947, w6946, w6945, w6941, w6941, w6941, FALSE, w6944) -> (w6943:bool[])
          }
        }
        "CH2_CH_VBV_DI" <- w6897
        "CH2_PL_VBV_DI" <- w6896
        n4213 = call "MB Serial Master Query Write Multiple Coils (poly).vi"("VISA resource name"=w6902, "Starting Address"=u16 320, "Coils"=w6906, "error in"=w6901, "Serial Parameters"=T15 {"Mode"=enum."RTU", "Slave Address"=1}) -> ("VISA resource name out"=w6908:refnum<visa-resource-name>, "error out"=w6907:errorcluster)  [unwired: 12 in, 1 out]
        n4214 = local read "CH2 I/O Loading"() -> (w6903:bool)
        n4215 = case shown="False" w6903 {
          tunnel: [w6914 w6923] -> w6905
          tunnel: ["CH2_SoV_Ar_DO" w6922] -> w6898
          frame False {
            n4216 = Build Array("CH2_SoV_Ar_DO", "CH2_Trns_GV_Open_DO", "CH2_Trns_GV_Close_DO", "CH2_Trns_BP_Right_DO", "CH2_Cst_Fix_DO", "CH2_M2_D6_DO", "CH2_PetCool_Up_DO", "CH2_PetCool_Down_DO") -> (w6914:bool[])
          }
          frame True {
            w6922 = FALSE
            n4217 = local read "CH2_PetCool_Down_DI"() -> (w6926:bool)
            n4218 = local read "CH2_Trns_Gv_Open_DI"() -> (w6930:bool)
            n4219 = local read "CH2_Trns_Gv_Close_DI"() -> (w6929:bool)
            n4220 = local read "CH2_Cst_Fix_Down_DI"() -> (w6927:bool)
            n4221 = local read "CH2_PetCool_Up_DI"() -> (w6925:bool)
            n4222 = local read "CH2_Trns_BP_Right_DI"() -> (w6928:bool)
            n4223 = Build Array(w6922, w6930, w6929, w6928, w6927, FALSE ("element"), w6925, w6926) -> (w6923:bool[])
          }
        }
        "CH2_SoV_Ar_DI" <- w6898
        n4224 = call "MB Serial Master Query Write Multiple Coils (poly).vi"("VISA resource name"=w6908, "Starting Address"=u16 320, "Coils"=w6905, "error in"=w6907, "Serial Parameters"=T15 {"Mode"=enum."RTU", "Slave Address"=2}) -> ("VISA resource name out"=w6899:refnum<visa-resource-name>, "error out"=w6900:errorcluster)  [unwired: 12 in, 1 out]
      }
      frame #4 {
        # "CH2 DO 3&4"
        n4225 = local read "CH2 I/O Loading"() -> (w6953:bool)
        n4226 = case shown="False" w6953 {
          tunnel: [w6975 w6991] -> w6955
          frame False {
            n4227 = Build Array("CH2_SRV1_Piston_For_DO", "CH2_SRV1_Piston_Back_DO", "CH2_M3_D3_DO", "CH2_SRV_Direction_Clockwise_DO", "CH2_M3_D5_DO", "CH2_M3_D6_DO", "CH2_WFC_DO", "CH2_Trns_BP_Left_DO") -> (w6975:bool[])
          }
          frame True {
            w6984 = FALSE
            n4228 = local read "CH2_SRV1_Piston_Back_DI"() -> (w6989:bool)
            n4229 = local read "CH2_SRV1_Piston_For_DI"() -> (w6990:bool)
            n4230 = local read "CH2_Trns_BP_Left_DI"() -> (w6986:bool)
            n4231 = local read "CH2_M3_D6_DI"() -> (w6988:bool)
            n4232 = local read "CH2_WFC_DI"() -> (w6987:bool)
            n4233 = Build Array(w6990, w6989, w6984, w6984, FALSE, w6988, w6987, w6986) -> (w6991:bool[])
          }
        }
        n4234 = call "MB Serial Master Query Write Multiple Coils (poly).vi"("VISA resource name"=w6951, "Starting Address"=u16 320, "Coils"=w6955, "error in"=w6950, "Serial Parameters"=T15 {"Mode"=enum."RTU", "Slave Address"=3}) -> ("VISA resource name out"=w6957:refnum<visa-resource-name>, "error out"=w6956:errorcluster)  [unwired: 12 in, 1 out]
        n4235 = local read "CH2 I/O Loading"() -> (w6952:bool)
        n4236 = case shown="False" w6952 {
          tunnel: [w6962 w6974] -> w6954
          frame False {
            n4237 = Build Array("CH2_LN2_DO", "CH2_M4_D2_DO", "CH2_TGV_Control_DO", "CH2_M4_D4_DO", "CH2_Right_Limit_DO", "CH2_Right_Slow_DO", "CH2_Left_Slow_DO", "CH2_Left_Limit_DO") -> (w6962:bool[])
          }
          frame True {
            w6971 = FALSE
            w6973 = FALSE
            n4238 = local read "CH2_TGV_Control_DI"() -> (w6972:bool)
            n4239 = Build Array(w6973, w6973, w6972, w6971, w6971, w6971, w6971, w6971) -> (w6974:bool[])
          }
        }
        n4240 = call "MB Serial Master Query Write Multiple Coils (poly).vi"("VISA resource name"=w6957, "Starting Address"=u16 320, "Coils"=w6954, "error in"=w6956, "Serial Parameters"=T15 {"Mode"=enum."RTU", "Slave Address"=4}) -> ("VISA resource name out"=w6948:refnum<visa-resource-name>, "error out"=w6949:errorcluster)  [unwired: 12 in, 1 out]
      }
      frame #5 {
        # "CH2 AI&AO"
        n4241 = call "MB Serial Master Query Read Input Registers (poly).vi"("VISA resource name"=w7010, "Starting Address"=u16 704 ("Quantity"), "Quantity"=u16 8, "error in"=w7009, "Serial Parameters"=T15 {"Mode"=enum."RTU", "Slave Address"=5}) -> ("VISA resource name out"=w7008:refnum<visa-resource-name>, "Input Registers"=w7021:u16[], "error out"=w7007:errorcluster)  [unwired: 11 in, 1 out]
        n4242 = Index Array(array=w7021, index #1=0 ("index"), index #2=1 ("index"), index #3=2 ("index"), index #4=3 ("index"), index #5=4 ("index"), index #6=5 ("index"), index #7=6 ("index"), index #8=7 ("index")) -> (element #1=→"CH2_Ai_Pl_Pg":u16, element #2=→"CH2_Ai_Ch_Pg":u16, element #3=→"CH2_Ai_Ch_Cc":u16, element #4=→"CH2_Ai_A4":u16, element #5=→"CH2_Ai_A5":u16, element #6=→"CH2_Ai_A6":u16, element #7=→"CH2_LN2_TK_t":u16, element #8=→"CH2_LN2_TK_b":u16)
        n4243 = Build Array(FALSE, "CH2 AO1 Set", "CH2 AO2 Set", "CH2 AO3 Set", "CH2 AO4 Set") -> (w7000:bool[])
        n4244 = Boolean Array To Number(Boolean array=w7000) -> (number=w7001:u32)
        n4245 = Mantissa & Exponent(0:w7001) -> (2:w6994:dbl)  [unwired: 1 out]
        n4246 = case shown="2" w6994 {
          tunnel: [0.0 ("TC2_Set_Value") "CH2 AO1" "CH2 AO2" "CH2 AO3" "CH2 AO4"] -> w7003
          tunnel: [0 1184 1185 1186 1187] -> w7002
          frame 0, Default {
          }
          frame 1 {
            n4247 = local write "CH2 AO1 Set"(FALSE ("CH1 AO1 Set")) -> ()
          }
          frame 2 {
            n4248 = local write "CH2 AO2 Set"(FALSE ("CH1 AO2 Set")) -> ()
          }
          frame 3 {
            n4249 = local write "CH2 AO3 Set"(FALSE ("CH1 AO3 Set")) -> ()
          }
          frame 4 {
            n4250 = local write "CH2 AO4 Set"(FALSE ("CH2 AO4 Set")) -> ()
          }
        }
        n4251 = Build Array(w7003) -> (w7004:dbl[])
        n4252 = call "MB Serial Master Query Write Multiple Registers (poly).vi"("VISA resource name"=w7008, "Starting Address"=w7002, "Registers"=w7004, "error in"=w7007, "Serial Parameters"=T15 {"Mode"=enum."RTU", "Slave Address"=6}) -> ("VISA resource name out"=w7006:refnum<visa-resource-name>, "error out"=w7005:errorcluster)  [unwired: 12 in, 1 out]
      }
      frame #6 {
      }
      frame #7 {
      }
    }
  }
  n4253 = while {
    tunnel: w35 -> [w7083]
    tunnel: w34 -> [w7082]
    tunnel: [w7066] -> w33
    tunnel: [w7065] -> w32
    stop <- FALSE stop-if-true
    n4254 = call "MB Serial Master Query Read Discrete Inputs (poly).vi"("VISA resource name"=w7083, "Starting Address"=u16 0 ("Quantity"), "Quantity"=u16 8, "error in"=w7082, "Serial Parameters"=T15 {"Mode"=enum."RTU", "Slave Address"=4}) -> ("VISA resource name out"=w7070:refnum<visa-resource-name>, "Discrete Inputs"=w7084:bool[], "error out"=w7069:errorcluster)  [unwired: 11 in, 1 out]
    n4255 = Index Array(array=w7084, index #1=0 ("index"), index #2=1 ("index"), index #3=2 ("index"), index #4=3 ("index"), index #5=4 ("index"), index #6=5 ("index"), index #7=6 ("index"), index #8=7 ("index")) -> (element #1=→"Ch1_srv1_counter DI":bool, element #2=→"Ch2_srv1_counter DI":bool, element #3=→"Ch3_srv1_counter DI":bool, element #4=→"Ch4_srv1_counter DI":bool, element #5=→"Center_4 DI5":bool, element #6=→"Center_4 DI6":bool, element #7=→"Center_4 DI7":bool, element #8=w7044:bool)
    "element" <- w7044
    n4256 = Wait Until Next ms Multiple(millisecond multiple=u32 100) -> ()  [unwired: 1 out]
    n4257 = feedback-in #137(w7044) -> ()
    n4258 = feedback #137() -> (w7057:bool)  [unwired: 1 in]
    n4259 = Boolean To (0,1)(Boolean=w7044) -> (0, 1=w7056:i16)
    n4260 = feedback #138() -> (w7051:bool)  [unwired: 1 in]
    n4261 = feedback-in #138(w7057) -> ()
    n4262 = Boolean To (0,1)(Boolean=w7057) -> (0, 1=w7055:i16)
    n4263 = Boolean To (0,1)(Boolean=w7051) -> (0, 1=w7054:i16)
    n4264 = feedback #139() -> (w7049:bool)  [unwired: 1 in]
    n4265 = feedback-in #139(w7051) -> ()
    n4266 = Boolean To (0,1)(Boolean=w7049) -> (0, 1=w7050:i16)
    n4267 = feedback #140() -> (w7047:bool)  [unwired: 1 in]
    n4268 = feedback-in #140(w7049) -> ()
    n4269 = Boolean To (0,1)(Boolean=w7047) -> (0, 1=w7048:i16)
    n4270 = feedback #141() -> (w7045:bool)  [unwired: 1 in]
    n4271 = feedback-in #141(w7047) -> ()
    n4272 = Boolean To (0,1)(Boolean=w7045) -> (0, 1=w7046:i16)
    n4273 = Compound Arithmetic op=ADD(w7056, w7055, w7054, w7050, w7048, w7046) -> (w7053:i16)
    n4274 = Greater?(x=w7053, y=i16 0) -> ()  [unwired: 1 out]
    n4275 = Build Array("CH1_Motor DO", "CH2_Motor DO", "CH3_Motor DO", "CH4_Motor DO") -> (w7071:bool[])
    n4276 = call "MB Serial Master Query Write Multiple Coils (poly).vi"("VISA resource name"=w7070, "Starting Address"=u16 320, "Coils"=w7071, "error in"=w7069, "Serial Parameters"=T15 {"Mode"=enum."RTU", "Slave Address"=4}) -> ("VISA resource name out"=w7066:refnum<visa-resource-name>, "error out"=w7065:errorcluster)  [unwired: 12 in, 1 out]
  }
  n4277 = while {
    tunnel: w99 -> [w7095]
    tunnel: w100 -> [w7094]
    tunnel: [w7092] -> w101
    tunnel: [w7093] -> w102
    stop <- FALSE stop-if-true
    n4278 = stacked-sequence {
      seq-local: [w7100 _ _ _] -> [_ w7369 _ _]
      seq-local: [w7101 _ _ _] -> [_ w7366 _ _]
      seq-local: [_ w7368 _ _] -> [_ _ w7608 _]
      seq-local: [_ w7367 _ _] -> [_ _ w7611 _]
      seq-local: [_ _ w7609 _] -> [_ _ _ w7874]
      seq-local: [_ _ w7610 _] -> [_ _ _ w7875]
      tunnel: w7095 -> [w7125 _ _ _]
      tunnel: w7094 -> [w7124 _ _ _]
      tunnel: [_ _ _ w7877] -> w7093
      tunnel: [_ _ _ w7876] -> w7092
      frame #0 {
        n4279 = Or(x="pcgv1 set position", y="pcgv1 auto set position") -> (x .or. y?=w7111:bool)
        n4280 = Compound Arithmetic op=OR("pcgv1 open gui 2", "pcgv1 auto open", "pcgv1 open gui", "pcgv1 open gui 1") -> (w7106:bool)
        n4281 = Compound Arithmetic op=OR("pcgv1 close gui 2", "pcgv1 close gui", "pcgv1 auto close", "pcgv1 close gui 1") -> (w7102:bool)
        n4282 = Or(x="pcgv1 set pressure gui", y="pcgv1 auto set pressure") -> (x .or. y?=w7113:bool)
        n4283 = Or(x="Baratron1 set zero gui", y="Baratron1 auto set zero") -> (x .or. y?=w7112:bool)
        n4284 = Build Array(FALSE, w7106, w7102, w7111, w7113, w7112, "Learn") -> (w7121:bool[])
        n4285 = Boolean Array To Number(Boolean array=w7121) -> (number=w7122:u32)
        n4286 = Mantissa & Exponent(0:w7122) -> (2:w7120:dbl)  [unwired: 1 out]
        n4287 = case shown="0, Default" w7120 {
          tunnel: w7125 -> [w7129 w7212 w7236 w7273 w7309 w7333 w7357]
          tunnel: w7124 -> [w7128 w7211 w7235 w7272 w7308 w7332 w7356]
          tunnel: [w7126 w7196 w7220 w7244 w7284 w7317 w7341] -> w7100
          tunnel: [w7127 w7195 w7219 w7243 w7283 w7316 w7340] -> w7101
          frame 0, Default {
            n4288 = stacked-sequence {
              seq-local: [w7132 _ _ _] -> [_ _ w7170 _]
              seq-local: [w7131 _ _ _] -> [_ _ w7169 _]
              tunnel: w7129 -> [w7147 _ _ _]
              tunnel: w7128 -> [w7146 _ _ _]
              tunnel: [_ _ w7168 _] -> w7127
              tunnel: [_ _ w7167 _] -> w7126
              frame #0 {
                n4289 = Concatenate Strings("#001A:" ("string"), "\r", "\n") -> (w7149:string)
                n4290 = VISA Write(VISA resource name=w7147, write buffer=w7149, error in (no error)=w7146) -> (VISA resource name out=w7145:refnum<visa-resource-name>, error out=w7144:errorcluster)  [unwired: 1 out]
                n4291 = stacked-sequence {
                  tunnel: [w7154] -> w7143
                  tunnel: w7145 -> [w7154]
                  tunnel: [w7153] -> w7142
                  tunnel: w7144 -> [w7153]
                  frame #0 {
                    n4292 = Wait (ms)(milliseconds to wait=u32 50) -> ()  [unwired: 1 out]
                  }
                }
                n4293 = property class="Instr"(reference=w7143, error in=w7142) -> (reference out=w7139:refnum<visa-resource-name>, error out=w7141:errorcluster, "Serial Settings:Number of Bytes at Serial Port"=w7140:u32)
                n4294 = VISA Read(VISA resource name=w7139, byte count=w7140, error in (no error)=w7141) -> (VISA resource name out=w7132:refnum<visa-resource-name>, read buffer=w7130:string, error out=w7131:errorcluster)  [unwired: 1 out]
                n4295 = Match Pattern(string=w7130, regular expression="#001A:") -> (after substring=w7137:string)  [unwired: 1 in, 3 out]
                n4296 = String Subset(string=w7137, offset (0)=0, length (rest)=3 ("length (rest)")) -> (substring=w7134:string)
                n4297 = Decimal String To Number(string=w7134) -> (number=→"pcgv1 position":i32)  [unwired: 2 in, 1 out]
              }
              frame #1 {
                n4298 = Wait (ms)(milliseconds to wait=u32 10) -> ()  [unwired: 1 out]
              }
              frame #2 {
                n4299 = Concatenate Strings("#001P:" ("string"), "\r", "\n") -> (w7186:string)
                n4300 = VISA Write(VISA resource name=w7170, write buffer=w7186, error in (no error)=w7169) -> (VISA resource name out=w7185:refnum<visa-resource-name>, error out=w7184:errorcluster)  [unwired: 1 out]
                n4301 = stacked-sequence {
                  tunnel: [w7193] -> w7183
                  tunnel: w7185 -> [w7193]
                  tunnel: [w7192] -> w7182
                  tunnel: w7184 -> [w7192]
                  frame #0 {
                    n4302 = Wait (ms)(milliseconds to wait=u32 50) -> ()  [unwired: 1 out]
                  }
                }
                n4303 = property class="Instr"(reference=w7183, error in=w7182) -> (reference out=w7179:refnum<visa-resource-name>, error out=w7181:errorcluster, "Serial Settings:Number of Bytes at Serial Port"=w7180:u32)
                n4304 = VISA Read(VISA resource name=w7179, byte count=w7180, error in (no error)=w7181) -> (VISA resource name out=w7167:refnum<visa-resource-name>, read buffer=w7172:string, error out=w7168:errorcluster)  [unwired: 1 out]
                n4305 = Match Pattern(string=w7172, regular expression="#001P:") -> (after substring=w7164:string)  [unwired: 1 in, 3 out]
                n4306 = String Subset(string=w7164, offset (0)=0, length (rest)=1 ("length (rest)")) -> (substring=w7163:string)
                n4307 = String Subset(string=w7164, offset (0)=2, length (rest)=4 ("length (rest)")) -> (substring=w7175:string)
                n4308 = Equal?(x=w7163, y="-") -> (x = y?=w7161:bool)
                n4309 = Decimal String To Number(string=w7175) -> (number=w7174:i32)  [unwired: 2 in, 1 out]
                n4310 = case shown="True" w7161 {
                  frame False {
                  }
                  frame True {
                    w7189 = u16 0 ("Ch1_baratron_pressure_mbar")
                    w7190 = 0.0 ("Pressure")
                    n4311 = local write "Pressure"(w7190) -> ()
                    n4312 = local write "Pressure_gui"(w7190) -> ()
                    n4313 = local write "Pressure_gui 2"(w7190) -> ()
                    n4314 = local write "Ch1_baratron_pressure_mbar 3"(w7189) -> ()
                    n4315 = local write "Ch1_baratron_pressure_mbar 2"(w7189) -> ()
                    n4316 = local write "Ch1_baratron_pressure_mbar"(w7189) -> ()
                  }
                }
                n4317 = Divide(x=w7174, y=100) -> (x/y=w7160:dbl)
                "Pressure" <- w7160
                "Pressure_gui" <- w7160
                "Pressure_gui 2" <- w7160
                n4318 = Multiply(x=w7160, y=0.00133) -> (x*y=w7156:dbl)
                "Ch1_baratron_pressure_mbar" <- w7156
                "Ch1_baratron_pressure_mbar 2" <- w7156
                "Ch1_baratron_pressure_mbar 3" <- w7156
                n4319 = Number To Exponential String(number=w7156, precision (6)=i16 3) -> (E-format string=→"CH1 CH BG":string)  [unwired: 2 in]
              }
              frame #3 {
                n4320 = Wait (ms)(milliseconds to wait=u32 10) -> ()  [unwired: 1 out]
              }
            }
          }
          frame 1 {
            n4321 = Concatenate Strings("#001O:" ("string"), "\r", "\n") -> (w7208:string)
            n4322 = VISA Write(VISA resource name=w7212, write buffer=w7208, error in (no error)=w7211) -> (VISA resource name out=w7200:refnum<visa-resource-name>, error out=w7199:errorcluster)  [unwired: 1 out]
            n4323 = local write "pcgv1 auto open"(FALSE ("Pc_bv1_auto_open")) -> ()
            n4324 = stacked-sequence {
              tunnel: [w7218] -> w7205
              tunnel: w7200 -> [w7218]
              tunnel: [w7217] -> w7204
              tunnel: w7199 -> [w7217]
              frame #0 {
                n4325 = Wait (ms)(milliseconds to wait=u32 50) -> ()  [unwired: 1 out]
              }
            }
            n4326 = property class="Instr"(reference=w7205, error in=w7204) -> (reference out=w7201:refnum<visa-resource-name>, error out=w7203:errorcluster, "Serial Settings:Number of Bytes at Serial Port"=w7202:u32)
            n4327 = VISA Read(VISA resource name=w7201, byte count=w7202, error in (no error)=w7203) -> (VISA resource name out=w7198:refnum<visa-resource-name>, error out=w7197:errorcluster)  [unwired: 2 out]
            n4328 = stacked-sequence {
              tunnel: [w7215] -> w7196
              tunnel: w7198 -> [w7215]
              tunnel: [w7214] -> w7195
              tunnel: w7197 -> [w7214]
              frame #0 {
                n4329 = Wait (ms)(milliseconds to wait=u32 50) -> ()  [unwired: 1 out]
              }
            }
          }
          frame 2 {
            n4330 = Concatenate Strings("#001C:" ("string"), "\r", "\n") -> (w7232:string)
            n4331 = local write "pcgv1 auto close"(FALSE ("Pc_bv1_auto_close")) -> ()
            n4332 = VISA Write(VISA resource name=w7236, write buffer=w7232, error in (no error)=w7235) -> (VISA resource name out=w7221:refnum<visa-resource-name>, error out=w7222:errorcluster)  [unwired: 1 out]
            n4333 = stacked-sequence {
              tunnel: [w7242] -> w7229
              tunnel: w7221 -> [w7242]
              tunnel: [w7241] -> w7228
              tunnel: w7222 -> [w7241]
              frame #0 {
                n4334 = Wait (ms)(milliseconds to wait=u32 50) -> ()  [unwired: 1 out]
              }
            }
            n4335 = property class="Instr"(reference=w7229, error in=w7228) -> (reference out=w7225:refnum<visa-resource-name>, error out=w7227:errorcluster, "Serial Settings:Number of Bytes at Serial Port"=w7226:u32)
            n4336 = VISA Read(VISA resource name=w7225, byte count=w7226, error in (no error)=w7227) -> (VISA resource name out=w7224:refnum<visa-resource-name>, error out=w7223:errorcluster)  [unwired: 2 out]
            n4337 = stacked-sequence {
              tunnel: [w7239] -> w7220
              tunnel: w7224 -> [w7239]
              tunnel: [w7238] -> w7219
              tunnel: w7223 -> [w7238]
              frame #0 {
                n4338 = Wait (ms)(milliseconds to wait=u32 50) -> ()  [unwired: 1 out]
              }
            }
          }
          frame 3 {
            n4339 = In Range and Coerce(upper limit=100.0, x="pcgv1 set position value", lower limit=0.0) -> (coerced(x)=w7263:dbl)  [unwired: 1 out]
            n4340 = Multiply(x=w7263, y=1000.0) -> (x*y=w7260:dbl)
            n4341 = Number To Decimal String(number=w7260) -> (decimal integer string=w7261:string)  [unwired: 1 out]